vi "UHR-Fleezers Control (host) - 12.0.vi"() -> ()   [LabVIEW 2014] (continued)
  T41 = enum32{"Normal Display", "Dual Display (APD)", "FFT", "High Res Display"}
  T42 = cluster{"Origin Pixel":cluster{"X":sgl, "Y":sgl}, "Angle Relative to Horizontal (deg)":sgl, "Axis Reference":u32}
  T43 = typedef "Simple Grid Descriptor" = cluster{"X Step":sgl, "Y Step":sgl, "Unit":T44}
  T44 = typedef "Image Unit" = enum32{"Undefined", "Angström", "Micrometer", "Millimeter", "Centimeter", "Meter", "Kilometer", "Microinch", "Inch", "Feet", "Nautical miles", "Standard miles", "Steps"}
  T45 = cluster{"averaging mode":u16, "weighting mode":u16, "number of averages":u32}
  T46 = cluster{"dB On (F)":bool, "unwrap phase (F)":bool, "convert to degree (F)":bool}
  T47 = cluster{string, string, string, string, string, string, string, string}
  T48 = cluster{string, string, string, string, string, string, string, string, string, string, string, string}
  T49 = cluster{string, string, string, string, string, string, string, string, string, string, string, string, string}
  T50 = cluster{string, string, string, string, string, string, string, string, string, string, string, string, string, string}
  T51 = cluster{"BD 1 Frequency 1 (MHz)":dbl, "BD 1 Frequency 2 (MHz)":dbl}
  T52 = cluster{"f0":dbl, "df":dbl, "magnitude":dbl[]}[][]
diagram:
  w11 = T19 1073684535 items=["Service Request"=1073684491, "Trigger"=3221168138, "Clear"=1073684493, "VXI Signal"=1073684512, "VXI/VME Interrupt"=3221168161, "VXI/VME Sysfail"=1073684509, "VXI/VME Sysreset"=1073684510, "GPIB CIC"=1073684498, "GPIB Talk"=1073684499, "GPIB Listen"=1073684500, "PXI Interrupt"=1073684514, "Serial Break"=1073684515, "Serial TermChar"=1073684516, "Serial CTS"=1073684521, "Serial DSR"=1073684522, "Serial DCD"=1073684524, "Serial RI"=1073684526, "Serial Character"=1073684533, "USB Interrupt"=1073684535, "All Enabled"=1073709055] ("Event Type")
  w45 = 0.0 ("Total Volume\nFlowed P1 (uL)")
  w57 = u16 20 items=["1.0"=10, "1.5"=15, "2.0"=20] ("stop bits (10: 1 bit)")
  w60 = u16 20 items=["1.0"=10, "1.5"=15, "2.0"=20] ("stop bits (10: 1 bit)")
  w114 = u16 20 items=["1.0"=10, "1.5"=15, "2.0"=20] ("stop bits (10: 1 bit)")
  w121 = T20 2 items=["Grayscale (U8)", "Grayscale (I16)", "Grayscale (SGL)", "Complex (CSG)", "RGB (U32)", "HSL (U32)", "RGB (U64)", "Grayscale (U16)"] ("Image Type")
  w179 = cluster{"output high":i16, "output low":i16} {"output high"=3000, "output low"=0} ("FB output range 1")
  w250 = 10.0 ("y")
  w249 = 32767.0 ("y")
  w265 = 6.0  # clock mult.
  w266 = 49152000.0  # TCXO frequ.
  # "Open the RAW resource"
  # "Enable USB Interrupt Event"
  # "Safety limits on RF frequencies and amplitudes (for AOM protection)"
  # "Bottom 1 Harvard"
  # "Top 3 Harvard"
  # "Center Harvard"
  # "Bottom 1 Harvard"
  # "Top 3 Harvard"
  # "Center Harvard"
  n1 = Build Array("DIO count 1 (ticks)", "DIO count 2 (ticks)", "DIO count 3 (ticks)") -> (w166:u32[])
  n2 = local read "AO1"() -> (w244:dbl)
  n3 = local read "AO2"() -> (w243:dbl)
  n4 = local read "Scan Increment (MHz)"() -> (w261:dbl)
  n5 = local read "Continuous MCL Scanning"() -> (w231:bool)
  n6 = local read "Fast Scan Dir"() -> (w230:bool)
  n7 = local read "Number of scans (MCL)"() -> (w232:u64)
  n8 = property on="AI Count (ticks)" class="DigNum (strict)"("Val(Sgnl)"="AI Count (ticks)") -> ()  [unwired: 2 in, 2 out]
  n9 = Multiply(x=w244, y=w249) -> (x*y=w246:dbl)
  n10 = Multiply(x=w243, y=w249) -> (x*y=w248:dbl)
  n11 = Divide(x=w246, y=w250) -> (x/y=w245:dbl)
  n12 = Divide(x=w248, y=w250) -> (x/y=w247:dbl)
  n13 = To Word Integer(number=w245) -> (16bit integer=w242:i16)
  n14 = To Word Integer(number=w247) -> (16bit integer=w241:i16)
  n15 = Not(x=w230) -> (.not. x?=w225:bool)
  n16 = local read "Cycles/step (MCL)"() -> (w233:u64)
  n17 = Multiply(x=w261, y=1000.0) -> (x*y=w268:dbl)
  n18 = local read "Scan steps (MCL)"() -> (w234:u64)
  n19 = local write "Trap Pos FIFO Timeout"(u16 0 ("Trap Pos FIFO Timeout")) -> ()
  n20 = local read "Desired Scan Incr (V)"() -> (w236:dbl)
  n21 = Scale By Power Of 2(n=48, x=w268) -> (x*2^n=w269:dbl)
  n22 = Multiply(x=w266, y=w265) -> (x*y=w264:dbl)
  n23 = Divide(x=w269, y=w264) -> (x/y=w263:dbl)
  n24 = local read "Setpoints (V)"() -> (w280:cluster{"Set 1":dbl, "Set 2":dbl})
  n25 = To Quad Integer(1:w263) -> (0:w260:i64)
  n26 = Divide(x=40000000.0, y="AI Count (ticks)") -> (x/y=w221:dbl)
  n27 = Multiply(x=w236, y=32767.0) -> (x*y=w238:dbl)
  n28 = local read "Number Interlace Sets"() -> (w159:u8)
  n29 = Split 1D Array(array=w166, index=w159) -> (first subarray=w168:u32[])  [unwired: 1 out]
  n30 = Add Array Elements(numeric array=w168) -> (sum=w167:u32)
  n31 = local read "# Samples/channel"() -> (w253:u32)
  n32 = local read "Number of F/B Scans (AOD)"() -> (w254:u16)
  n33 = local read "Not-Interlacing Set"() -> (w158:enum32{"Set 1", "Set 2", "Set 3"})
  n34 = To Unsigned Byte Integer(number=w158) -> (unsigned 8bit integer=w164:u8)
  n35 = Index Array(array=w166, index=w164) -> (element=w165:u32)
  n36 = local read "Feedback On/Off"() -> (w283:cluster{"Set 1":bool, "Set 2":bool})
  n37 = local read "PID Gains"() -> (w275:T9)
  n38 = local read "Scan steps (AOD)"() -> (w259:u64)
  n39 = local read "All FB On/Off"() -> (w284:bool)
  n40 = local read "Cycles/step (AOD)"() -> (w258:u64)
  n41 = local write "AI rate (Hz)"(w221) -> ()
  n42 = Divide(x=w238, y=10.0) -> (x/y=w237:dbl)
  n43 = Multiply(x=w259, y=w258) -> (x*y=w257:u64)
  n44 = Multiply(x=3276.7, y=w280) -> (x*y=w279:cluster{"Set 1":dbl, "Set 2":dbl})
  n45 = To Word Integer(number=w237) -> (16bit integer=w235:i16)
  n46 = xnode "Open FPGA VI Reference"("resource name"=T21 "RIO1") -> ("FPGA VI Reference Out"=w43:T22, "error out"=w41:errorcluster)  [unwired: 1 in]
  n47 = Multiply(x=w257, y=u64 2) -> (x*y=w255:u64)
  n48 = local read "Sets to FIFO (Traps)"() -> (w287:T16)
  n49 = Divide(x=w221, y="FPGA Ave.") -> (x/y=w222:dbl)
  n50 = To Word Integer(number=w279) -> (16bit integer=w278:cluster{"Set 1":i16, "Set 2":i16})
  n51 = Unbundle By Name(w275) -> ("Set 1"=w274:T15, "Set 2"=w273:T15)
  n52 = Multiply(x=w255, y=w254) -> (x*y=w252:u64)
  n53 = local write "Ave. Rate (Hz)"(w222) -> ()
  n54 = Divide(x=w252, y=w253) -> (x/y=w251:dbl)
  n55 = Unbundle By Name(w278) -> ("Set 1"=w277:i16, "Set 2"=w276:i16)
  n56 = local read "2D or 1D Scan"() -> (w180:bool)
  n57 = local write "Data points/scans"(w252) -> ()
  n58 = local read "Scan BD"() -> (w270:bool)
  n59 = And(x=w283, y=w284) -> (x .and. y?=w282:cluster{"Set 1":bool, "Set 2":bool})
  n60 = local write "Data points/scan (f/b)"(w255) -> ()
  n61 = Reciprocal(x=w222) -> (1/x=w223:dbl)
  n62 = local read "N Acq Sets (Traps + Fl.)"() -> (w214:i16)
  n63 = local write "N sets should be saved"(w251) -> ()
  n64 = xnode "Invoke Method"("FPGA VI Reference In"=w43, "error in"=w41) -> ("FPGA VI Reference Out"=w178:T22, "error out"=w188:errorcluster)
  n65 = Unbundle By Name(w282) -> ("Set 1"=w286:bool, "Set 2"=w285:bool)
  n66 = local read "Interlace"() -> (w160:bool)
  n67 = Select(t=w167, s=w160, f=w165) -> (s? t:f=w157:u32)
  n68 = local write "Update Count (MCL)"(w157) -> ()
  n69 = local write "Total Counts (ticks)"(w157) -> ()
  n70 = local write "Ave. Period (s)"(w223) -> ()
  n71 = property on="2D or 1D Scan" class="Bool (strict)"("Val(Sgnl)"=w180) -> ()  [unwired: 2 in, 2 out]
  n72 = local read "APD Gate OFF Count"() -> (w84:u16)
  n73 = local read "Interlace OFF count"() -> (w87:u16)
  n74 = local read "Interlace ON count"() -> (w22:u16)
  n75 = local read "APD Gate ON Count"() -> (w80:u16)
  n76 = xnode "Read/Write Control"("FPGA VI Reference In"=w177, "error in"=w188, "ai count"="AI Count (ticks)", "Interlace ON/OFF"=w160, "Number Interlace Cycles"=w159, "AI1 Sets to FIFO"=w287, "FB On/Off Set 1"=w286, "FB On/Off Set 2"=w285, "Interlace Off Parameters"=w158, "FB Setpoint Set 1"=w277, "FB Setpoint Set 2"=w276, "FB Gains Set 1"=w274, "FB Gains Set 2"=w273, "FB output range 1"=w179, "FB output range 2"=w179, "Cycles per step"=w258, "Scan BD"=w270, "Number of scans"=w254, "Scan steps"=w259, "Scan freq.  increment"=w260, "AO1"=w242, "AO2"=w241, "Scan freq.  increment (MCL)"=w235, "Scan steps (MCL)"=w234, "Cycles per step (MCL)"=w233, "Number of scans (MCL)"=w232, "MCL count"=w157, "Cont. Scan (MCL)"=w231, "MCL Scan Axis"=w225, "1D or 2D Scan?"=w180, "N of AI1 Int Acq Sets"=w214, "Freq or Amp switch first"="Freq or Amp switch first", "Freq switch delay"="Freq switch delay", "Amp switch delay"="Amp switch delay", "Swap F1 and F2"="Swap F1 and F2", "APD to FIFO"=FALSE, "DIO count 1 (ticks)"="DIO count 1 (ticks)", "DIO count 2 (ticks)"="DIO count 2 (ticks)", "DIO count 3 (ticks)"="DIO count 3 (ticks)") -> ("FPGA VI Reference Out"=w91:T22, "error out"=w89:errorcluster)  [unwired: 1 in]
  n77 = local read "Duty frequency (ON 1/N cycles)"() -> (w86:u16)
  n78 = local read "APD Integration Time (s)"() -> (w72:dbl)
  n79 = local read "DMA Update Period (s)"() -> (w71:dbl)
  n80 = local read "Red Laser ON/Interlacing"() -> (w25:bool)
  n81 = Add(x=w80, y=w84) -> (x+y=w82:u16)
  n82 = local read "Laser interlacing mode (all lasers)"() -> (w24:enum32{"Laser ON", "Laser OFF", "Interlace"})
  n83 = Add(x=w22, y=w87) -> (x+y=w85:u16)
  n84 = local read "Green ON/Interlacing"() -> (w156:bool)
  n85 = Multiply(x=w82, y=w86) -> (x*y=w83:u16)
  n86 = Multiply(x="Red FB Setpoint (mV)", y=3.2767) -> (x*y=w15:dbl)
  n87 = Multiply(x=w86, y=w85) -> (x*y=w79:u16)
  n88 = Reciprocal(x=w72) -> (1/x=w69:dbl)
  n89 = Multiply(x=w72, y=40000000.0) -> (x*y=w68:dbl)
  n90 = Divide(x=w71, y=w72) -> (x/y=w74:dbl)
  n91 = Multiply(x="Green intensity % (FB OFF)", y=655.35) -> (x*y=w146:dbl)
  n92 = local read "Invert laser interlacing"() -> (w20:bool)
  n93 = case shown="False" w25 {
    tunnel: w24 -> [_ w311]
    tunnel: [enum32{"Laser ON", "Laser OFF", "Interlace"}."Laser OFF" ("Laser interlacing mode (all lasers)") w311] -> w23
    frame False {
    }
    frame True {
    }
  }
  n94 = local read "Invert APD Gate"() -> (w78:bool)
  n95 = Multiply(x="Green FB Setpoint (mV)", y=3.2767) -> (x*y=w143:dbl)
  n96 = local read "APD Gate"() -> (w77:enum32{"ON", "OFF", "Interlace"})
  n97 = Subtract(x=w83, y=w80) -> (x-y=w81:u16)
  n98 = To Word Integer(number=w15) -> (16bit integer=w14:i16)
  n99 = local write "Green FB Count"(w79) -> ()
  n100 = local write "APD Acq Rate (Hz)"(w69) -> ()
  n101 = To Unsigned Long Integer(number=w68) -> (unsigned 32bit integer=w66:u32)
  n102 = Multiply(x=2.0, y=w74) -> (x*y=w73:dbl)
  n103 = To Unsigned Word Integer(number=w146) -> (unsigned 16bit integer=w144:u16)
  n104 = Subtract(x=w79, y=w22) -> (x-y=w21:u16)
  n105 = local write "APD Samples/FIFO Acq."(w74) -> ()
  n106 = To Word Integer(number=w143) -> (16bit integer=w141:i16)
  n107 = local write "APD Elements/DMA read"(w73) -> ()
  n108 = case shown="False" w156 {
    tunnel: w24 -> [_ w313]
    tunnel: [enum32{"Laser ON", "Laser OFF", "Interlace"}."Laser OFF" ("Green laser mode") w313] -> w26
    frame False {
    }
    frame True {
    }
  }
  n109 = local write "APD Int. Count"(w66) -> ()
  n110 = Multiply(x="Red intensity % (FB OFF)", y=655.35) -> (x*y=w30:dbl)
  n111 = local read "Trap Pos. AI1 X Pre-scale"() -> (w101:u16)
  n112 = local read "Trap Pos FB Monitor\nT1 or T2"() -> (w108:bool)
  n113 = To Unsigned Word Integer(number=w30) -> (unsigned 16bit integer=w29:u16)
  n114 = local read "Trap Pos FB Int Count"() -> (w95:u16)
  n115 = local read "APD 1 AO Mult."() -> (w76:i16)
  n116 = local read "Trap Pos FB Negate Action"() -> (w107:bool)
  n117 = local read "APD 2 AO Mult."() -> (w75:i16)
  n118 = local read "Trap Pos. FB Offset Factor"() -> (w106:i64)
  n119 = local read "Trap Pos. FB Mult Factor"() -> (w105:i64)
  n120 = local read "Differential FB?"() -> (w63:bool)
  n121 = local read "Neg. TTrig FPGA"() -> (w65:bool)
  n122 = local read "Trap Pos. FB Gains"() -> (w103:T11)
  n123 = local read "Trap Pos. FB Range"() -> (w104:T12)
  n124 = xnode "Read/Write Control"("FPGA VI Reference In"=w91, "error in"=w89, "Invert APD Gate"=w78, "APD Gate ON Count"=w80, "APD Gate OFF Count"=w81, "APD Acq Rate Count"=w66, "APD Gate Operating Mode"=w77, "APD 1 AO scale factor"=w76, "APD 2 AO scale factor"=w75, "Green interlace ON count"=w22, "Green interlace OFF count"=w21, "Green interlace ON count 2"=w22, "Green interlace OFF count 2"=w21, "Green FB Count"=w79, "RI ON count"=w22, "RI OFF count"=w21) -> ("FPGA VI Reference Out"=w90:T22, "error out"=w88:errorcluster)
  n125 = xnode "Read/Write Control"("FPGA VI Reference In"=w90, "error in"=w88, "Invert GI 2"=w20, "Operating Mode 2"=w26, "Green FB Gains"="Green FB Gains", "Green FB Setpoint"=w141, "Green FB On/Off"="Green FB On/Off", "Current Out"=w144, "Green int current ON count adj"="Green int current ON count adj", "Operating Mode"=w26, "Invert GI"=w20, "Trap Pos FB Monitor T1 or T2"=w108, "Trap Pos FB Negate Action"=w107, "Trap Pos. FB Offset Factor"=w106, "Trap Pos. FB Mult Factor"=w105, "Trap Pos. FB Range"=w104, "Trap Pos. FB Gains"=w103, "Force feedback"=FALSE, "AI1 X Scale"=w101, "Trap Pos to FIFO"=TRUE, "Trap Pos FB Int Count"=w95, "TTrig Negate Pos"=w65, "FB Trig Integrate"="FB Trig Integrate", "Diff FB Measurement?"=w63, "Negate Diff?"="Negate Diff?", "RI Current Out"=w29, "Red operating mode"=w23, "RI operating mode 2"=w23, "Invert RI"=w20, "Invert RI 2"=w20, "Red FB Gains"="Red FB Gains", "Red FB On/Off"="Red FB On/Off", "Red FB Setpoint"=w14) -> ("FPGA VI Reference Out"=w154:T22, "error out"=w155:errorcluster)
  n126 = xnode "Invoke Method"("FPGA VI Reference In"=w154, "error in"=w155, "Requested Depth"="Trap AI FIFO Depth") -> ("FPGA VI Reference Out"=w110:T22, "error out"=w109:errorcluster)  [unwired: 1 out]
  n127 = xnode "Invoke Method"("FPGA VI Reference In"=w110, "error in"=w109, "Requested Depth"="Trap Position FIFO Depth") -> ("FPGA VI Reference Out"=w97:T22, "error out"=w96:errorcluster)  [unwired: 1 out]
  n128 = flat-sequence {
    tunnel: w178 -> [w318]
    tunnel: [w318] -> w177
    tunnel: [w317] -> w176
    tunnel: [w316] -> w175
    tunnel: [w314] -> w173
    tunnel: [w315] -> w174
    frame #0 {
      w315 = T17 {"Minimum"=0.0, "Maximum"=40.0, "Increment"=1.0} ("Min Max Inc")
      w314 = T17 {"Minimum"=0.0, "Maximum"=50.0, "Increment"=1.0} ("Data Entry Limits")
      w317 = T17 {"Minimum"=60.0, "Maximum"=90.0, "Increment"=1.0} ("Min Max Inc")
      w316 = T17 {"Minimum"=0.0, "Maximum"=50.0, "Increment"=1.0} ("Data Entry Limits")
      n129 = property on="BD 2 Frequency 1 (MHz)" class="DigNum (strict)"("Data Range"=w315) -> ()  [unwired: 2 in, 2 out]
      n130 = property on="BD 2 Frequency 3 (MHz)" class="DigNum (strict)"("Data Range"=w315) -> ()  [unwired: 2 in, 2 out]
      n131 = property on="BD 2 Frequency 2 (MHz)" class="DigNum (strict)"("Data Range"=w315) -> ()  [unwired: 2 in, 2 out]
      n132 = property on="BD 1 Frequency 1 (MHz)" class="DigNum (strict)"("Data Range"=w317) -> ()  [unwired: 2 in, 2 out]
      n133 = property on="BD 1 Frequency 2 (MHz)" class="DigNum (strict)"("Data Range"=w317) -> ()  [unwired: 2 in, 2 out]
      n134 = property on="BD 1 Frequency 3 (MHz)" class="DigNum (strict)"("Data Range"=w317) -> ()  [unwired: 2 in, 2 out]
      n135 = property on="BD 2 Amplitude 1 (%)" class="DigNum (strict)"("Data Range"=w314) -> ()  [unwired: 2 in, 2 out]
      n136 = property on="BD 2 Amplitude 2 (%)" class="DigNum (strict)"("Data Range"=w314) -> ()  [unwired: 2 in, 2 out]
      n137 = property on="BD 2 Amplitude 3 (%)" class="DigNum (strict)"("Data Range"=w314) -> ()  [unwired: 2 in, 2 out]
      n138 = property on="BD 1 Amplitude 3 (%)" class="DigNum (strict)"("Data Range"=w316) -> ()  [unwired: 2 in, 2 out]
      n139 = property on="BD 1 Amplitude 2 (%)" class="DigNum (strict)"("Data Range"=w316) -> ()  [unwired: 2 in, 2 out]
      n140 = property on="BD 1 Amplitude 1 (%)" class="DigNum (strict)"("Data Range"=w316) -> ()  [unwired: 2 in, 2 out]
      "X RF Frequency Limits (MHz)" <- w317
      "X RF Amplitude Limits (%)" <- w316
      "Y RF Amplitude Limits (%)" <- w314
      "Y RF Frequency Limits (MHz)" <- w315
    }
  }
  n141 = xnode "Invoke Method"("FPGA VI Reference In"=w97, "error in"=w96) -> ("FPGA VI Reference Out"=w187:T22, "error out"=w186:errorcluster)  [unwired: 1 in]
  n142 = flat-sequence "Initial FPGA Loop Relative Phase Adjustment" {
    tunnel: "Initial Phase Adjustment (APD 2 Gate)" -> [w321]
    tunnel: "Initial Phase Adjust (GI) 2" -> [w322]
    tunnel: "Initial Phase Adj. (MCL)" -> [w320]
    tunnel: w186 -> [w323]
    tunnel: w187 -> [w324]
    tunnel: "Initial Phase Adjust (GI)" -> [w325]
    tunnel: "Initial Phase Adjustment (AI1)" -> [w326]
    tunnel: [w326] -> w40
    tunnel: [w325] -> w39
    tunnel: [w324] -> w38
    tunnel: [w323] -> w37
    tunnel: [w320] -> w36
    tunnel: [w322] -> w35
    tunnel: [w321] -> w34
    tunnel: [w339] -> w196
    tunnel: [w333] -> w192
    tunnel: "Initial Phase Adjustment (APD Acq)" -> [w332]
    tunnel: "Initial Phase Adjustment (APD 1 Gate)" -> [w331]
    tunnel: "Initial Phase Adjust (Green FB)" -> [w330]
    tunnel: w40 -> [w338]
    tunnel: w39 -> [w337]
    tunnel: w38 -> [w336]
    tunnel: w37 -> [w335]
    tunnel: w36 -> [w334]
    tunnel: w35 -> [w329]
    tunnel: w34 -> [w328]
    tunnel: "Initial Phase Adjustment (RI)" -> [w327]
    tunnel: w196 -> [w341]
    tunnel: [w342] -> w193
    tunnel: w192 -> [w342]
    tunnel: [w341] -> w191
    tunnel: w193 -> [w345]
    tunnel: w191 -> [w344]
    tunnel: [w347] -> w190
    tunnel: [w346] -> w189
    tunnel: [w349] -> w194
    tunnel: [w350] -> w195
    tunnel: w190 -> [w350]
    tunnel: w189 -> [w349]
    frame #0 {
      n143 = Wait (ms)(milliseconds to wait=u32 100) -> ()  [unwired: 1 out]
    }
    frame #1 {
      n144 = xnode "Read/Write Control"("FPGA VI Reference In"=w336, "error in"=w335, "Phase count adjustment"=w338, "Phase count adjustment (GI)"=w337, "Phase count adjustment (MCL)"=w334, "Phase Count Adjustment (APD Acq)"=w332, "Phase count adjustment (APD 1 Gate)"=w331, "Phase count adjustment (APD 2 Gate)"=w328, "Phase count adjustment (Green FB)"=w330, "Phase count adjustment (GI) 2"=w329, "Phase count adjustment (RI)"=w327) -> ("FPGA VI Reference Out"=w333:T22, "error out"=w339:errorcluster)
    }
    frame #2 {
      n145 = Wait (ms)(milliseconds to wait=u32 100) -> ()  [unwired: 1 out]
    }
    frame #3 {
      w343 = TRUE
      n146 = xnode "Read/Write Control"("FPGA VI Reference In"=w345, "error in"=w344, "+ phase"=w343, "+ phase (GI)"=w343, "+ phase (MCL)"=w343, "+ phase (APD Acq)"=w343, "+ phase (APD 1 Gate)"=w343, "+ phase (APD 2 Gate)"=w343, "+ phase (Green FB)"=w343, "+ phase (GI) 2"=w343, "+ phase (RI)"=w343) -> ("FPGA VI Reference Out"=w346:T22, "error out"=w347:errorcluster)
    }
    frame #4 {
      n147 = Wait (ms)(milliseconds to wait=u32 100) -> ()  [unwired: 1 out]
    }
  }
  n148 = VISA Open(VISA resource name="USB port") -> (VISA resource name=w13:refnum<visa-resource-name>, error out=w12:errorcluster)  [unwired: 1 in, 3 out]
  n149 = local read "Phase adj. (Green FB)"() -> (w169:i16)
  n150 = local read "Phase adj. (GI) 2"() -> (w147:i16)
  n151 = local read "Phase adj. (RI)"() -> (w27:i16)
  n152 = local read "Phase adjust (MCL)"() -> (w226:i16)
  n153 = local read "Phase adj. (AI1)"() -> (w228:i16)
  n154 = local read "Phase adj. (GI)"() -> (w227:i16)
  n155 = VISA Enable Event(8:w12, 10:w11, 11:w13) -> (0:w8:errorcluster, 3:w7:refnum<visa-resource-name>)  [unwired: 1 out]
  n156 = xnode "Read/Write Control"("FPGA VI Reference In"=w194, "error in"=w195, "Phase count adjustment"=w228, "Phase count adjustment (GI)"=w227, "Phase count adjustment (MCL)"=w226, "Phase Count Adjustment (APD Acq)"="Phase Adj. (APD Acq)", "Phase count adjustment (APD 1 Gate)"="Phase Adj. (APD 1 Gate)", "Phase count adjustment (APD 2 Gate)"="Phase Adj. (APD 2 Gate)", "Phase count adjustment (Green FB)"=w169, "Phase count adjustment (GI) 2"=w147, "Phase count adjustment (RI)"=w27) -> ("FPGA VI Reference Out"=w42:T22, "error out"=w203:errorcluster)
  n157 = call "Initialize RF boards - interlace 3.vi"("error in"=w203, "FPGA VI Reference In"=w42) -> ("error out"=w201:errorcluster, "FPGA VI Reference Out"=w202:T22)
  n158 = call "set RF board frequency - interlace.vi"("Board 2 Frequency Limits"=w174, "Board 1 Frequency Limits"=w176, "error in"=w201, "FPGA VI Reference In"=w202, "Board 2 Frequency 3 (MHz)"="BD 2 Frequency 3 (MHz)", "Board 1 Frequency 3 (MHz)"="BD 1 Frequency 3 (MHz)", "Board 2 Frequency 2 (MHz)"="BD 2 Frequency 2 (MHz)", "Board 2 Frequency 1 (MHz)"="BD 2 Frequency 1 (MHz)", "Board 1 Frequency 2 (MHz)"="BD 1 Frequency 2 (MHz)", "Board 1 Frequency 1  (MHz)"="BD 1 Frequency 1 (MHz)") -> ("error out"=w302:errorcluster, "FPGA VI Reference Out"=w303:T22)
  n159 = call "set RF board amplitude - interlace.vi"("Board 2 Amplitude Limits"=w173, "Board 1 Amplitude Limits"=w175, "error in"=w302, "FPGA VI Reference In"=w303, "Board 2 Amplitude 3 (%)"="BD 2 Amplitude 3 (%)", "Board 1 Amplitude 3 (%)"="BD 1 Amplitude 3 (%)", "Board 2 Amplitude 2 (%)"="BD 2 Amplitude 2 (%)", "Board 2 Amplitude 1 (%)"="BD 2 Amplitude 1 (%)", "Board 1 Amplitude 2 (%)"="BD 1 Amplitude 2 (%)", "Board 1 Amplitude 1 (%)"="BD 1 Amplitude 1 (%)") -> ("error out"=w290:errorcluster, "FPGA VI Reference Out"=w291:T22)
  n160 = flat-sequence {
    tunnel: w291 -> [w360]
    tunnel: w290 -> [w359]
    tunnel: [w358] -> w295
    tunnel: [w357] -> w294
    tunnel: [w364] -> w293
    tunnel: w295 -> [w364]
    tunnel: [w363] -> w292
    tunnel: w294 -> [w363]
    tunnel: w293 -> [w373]
    tunnel: w292 -> [w372]
    tunnel: [w371] -> w51
    tunnel: [w370] -> w98
    frame #0 {
      w351 = FALSE ("Retract Pump 3")
      n161 = local read "Trap 1 (ON/OFF)"() -> (w352:bool)
      n162 = xnode "Read/Write Control"("FPGA VI Reference In"=w360, "error in"=w359, "Direct RF Box  Communication"=FALSE) -> ("FPGA VI Reference Out"=w358:T22, "error out"=w357:errorcluster)
      n163 = local write "Saving..."(FALSE ("Saving Data")) -> ()
      n164 = local write "Stop All"(FALSE ("Stop All")) -> ()
      n165 = local write "Retract Pump 1"(w351) -> ()
      n166 = local write "Retract Pump 3"(w351) -> ()
      n167 = local write "Index"(1.0 ("Index")) -> ()
      n168 = property on="Trap 1 ON" class="Bool (strict)"("Value"=w352) -> ()  [unwired: 2 in, 2 out]
      "Manipulating Trap" <- FALSE ("Manipulating Trap")
    }
    frame #1 {
      n169 = local read "Trap 2 (ON/OFF)"() -> (w362:bool)
      n170 = Wait (ms)(milliseconds to wait=u32 10) -> ()  [unwired: 1 out]
      n171 = property on="Trap 2 ON" class="Bool (strict)"("Val(Sgnl)"=w362) -> ()  [unwired: 2 in, 2 out]
    }
    frame #2 {
      n172 = local read "Scan Range (nm)"() -> (w366:dbl)
      n173 = xnode "Read/Write Control"("FPGA VI Reference In"=w373, "error in"=w372, "FPGA Controls  RF Box"=TRUE ("Direct RF Box  Communication")) -> ("FPGA VI Reference Out"=w371:T22, "error out"=w370:errorcluster)
      n174 = call "Update messages.vi"("Message to add"="UHR-Fleezers ready.", "Old message string"="") -> ("New message string"=w369:string)
      n175 = local write "Messages"(w369) -> ()
      n176 = property on="Scan Range (nm)" class="DigNum (strict)"("Val(Sgnl)"=w366) -> ()  [unwired: 2 in, 2 out]
    }
  }
  n177 = Subtract(x="BD 1 Frequency 1 (MHz)", y="BD 1 Frequency 2 (MHz)") -> (x-y=w213:dbl)
  n178 = Subtract(x="BD 2 Frequency 1 (MHz)", y="BD 2 Frequency 2 (MHz)") -> (x-y=w212:dbl)
  n179 = Square(x=w212) -> (x^2=w210:dbl)
  n180 = Square(x=w213) -> (x^2=w211:dbl)
  n181 = Add(x=w211, y=w210) -> (x+y=w209:dbl)
  n182 = Square Root(x=w209) -> (sqrt(x)=w208:dbl)
  n183 = local write "Trap D (MHz)"(w208) -> ()
  n184 = call "IMAQ Create"("Image Name"="APD 1 Image", "Image Type"=w121) -> ("New Image"=w120:T2)  [unwired: 3 in, 1 out]
  n185 = call "IMAQ Create"("Image Name"="APD 2 Image", "Image Type"=w121) -> ("New Image"=w119:T2)  [unwired: 3 in, 1 out]
  n186 = call "IMAQ Create"("Image Name"="Det. X Image", "Image Type"=w121) -> ("New Image"=w118:T2)  [unwired: 3 in, 1 out]
  n187 = call "IMAQ Create"("Image Name"="Det. Y Image", "Image Type"=w121) -> ("New Image"=w117:T2)  [unwired: 3 in, 1 out]
  n188 = Bundle("New Image"=w120, "New Image"=w119, "New Image"=w118, "New Image"=w117) -> (w116:T23)  [unwired: 1 in]
  n189 = call-poly "VISA Configure Serial Port"("VISA resource name"="Bottom  1 Harvard Syringe Pump Serial Port", "baud rate (9600)"=u32 115200, "stop bits (10: 1 bit)"=w57) -> ("VISA resource name out"=w53:refnum<visa-resource-name>, "error out"=w52:errorcluster)  [unwired: 4 in, 7 out]
  n190 = call-poly "VISA Configure Serial Port"("VISA resource name"="Top 3 Harvard Syringe Pump Serial Port", "baud rate (9600)"=u32 115200, "stop bits (10: 1 bit)"=w60) -> ("VISA resource name out"=w55:refnum<visa-resource-name>, "error out"=w54:errorcluster)  [unwired: 4 in, 7 out]
  n191 = call-poly "VISA Configure Serial Port"("VISA resource name"="Sample Chamber Stage Serial Port", "baud rate (9600)"=u32 19200) -> ("VISA resource name out"=w5:refnum<visa-resource-name>, "error out"=w130:errorcluster)  [unwired: 4 in, 8 out]
  "Stage Control Serial Error" <- w130
  n192 = while {
    shift-right: [w393] -> w4
    shift-left: w8 -> [w394]
    shift-right: [w391] -> w3
    shift-left: w7 -> [w392]
    tunnel: w5 -> [w390]
    stop <- w395 stop-if-true
    n193 = global read "FAST_Global_var.vi" "FAST L"() -> (→"FAST Z" →"FAST Z":bool)
    n194 = global read "FAST_Global_var.vi" "FAST R"() -> (→"FAST X-Y" →"FAST X-Y":bool)
    n195 = call "LogitechSubVi.vi"("USB port"=w392, "VISA resource name in 2 (for the Newport)"=w390, "error in (no error)"=w394, "X-Y Wait time"="XY Wait time", "Z Wait time"="Z Wait time", "XY Speed Definitions"="XY Speed Definitions", "Z Speed Definitions"="Z Speed Definitions") -> ("Right stick button"=→"Right stick button":bool, "Left stick button"=→"Left stick button":bool, "USB port out"=w391:refnum<visa-resource-name>, "error out"=w393:errorcluster, "A B X Y"=w380:cluster{"A":bool, "B":bool, "X":bool, "Y":bool}, "LB RB"=w389:T24, "U D L R"=w381:cluster{"U":bool, "D":bool, "L":bool, "R":bool}, "Sticks"=w388:T25)  [unwired: 5 in]
    n196 = Unbundle By Name(w381) -> ("U"=→"U":bool, "D"=→"D":bool, "L"=→"L":bool, "R"=→"R":bool)
    n197 = Unbundle By Name(w389) -> ("LB"=w379:bool, "RB"=w378:bool, "BACK"=w376:bool, "Logitech"=w375:bool, "START"=w377:bool)
    "LB" <- w378
    "RB" <- w379
    "BACK" <- w376
    "START" <- w377
    "Logitech" <- w375
    n198 = case shown="True" w378 {
      frame False {
      }
      frame True {
        n199 = local read "Trap 1 (ON/OFF)"() -> (w424:bool)
        n200 = Not(x=w424) -> (.not. x?=w425:bool)
        n201 = property on="Trap 1 (ON/OFF)" class="Bool (strict)"("Val(Sgnl)"=w425) -> ()  [unwired: 2 in, 2 out]
      }
    }
    n202 = case shown="True" w376 {
      selector: w376 -> [_ w420]
      frame False {
      }
      frame True {
        n203 = property on="Move to Position 1" class="Bool (strict)"("Val(Sgnl)"=w420) -> ()  [unwired: 2 in, 2 out]
      }
    }
    n204 = case shown="True" w375 {
      frame False {
      }
      frame True {
        n205 = local read "Sample Channel\nFlow"() -> (w419:bool)
        n206 = Not(x=w419) -> (.not. x?=w418:bool)
        n207 = property on="Sample Channel\nFlow" class="Bool (strict)"("Val(Sgnl)"=w418) -> ()  [unwired: 2 in, 2 out]
      }
    }
    n208 = case shown="True" w379 {
      frame False {
      }
      frame True {
        n209 = local read "Trap 2 (ON/OFF)"() -> (w422:bool)
        n210 = Not(x=w422) -> (.not. x?=w423:bool)
        n211 = property on="Trap 2 (ON/OFF)" class="Bool (strict)"("Val(Sgnl)"=w423) -> ()  [unwired: 2 in, 2 out]
      }
    }
    n212 = case shown="True" w377 {
      selector: w377 -> [_ w421]
      frame False {
      }
      frame True {
        n213 = property on="Move to Position 2" class="Bool (strict)"("Val(Sgnl)"=w421) -> ()  [unwired: 2 in, 2 out]
      }
    }
    n214 = Unbundle By Name(w388) -> ("Right X"=w415:i8, "Right Y"=w414:i8, "Left X"=w412:i8, "Left Y"=w410:i8)
    n215 = Not Equal To 0?(x=w415) -> (x != 0?=w417:bool)
    n216 = Not Equal To 0?(x=w410) -> (x != 0?=w411:bool)
    n217 = Not Equal To 0?(x=w412) -> (x != 0?=w413:bool)
    n218 = Unbundle By Name(w380) -> ("A"=w402:bool, "B"=w400:bool, "X"=w398:bool, "Y"=w396:bool)
    "B" <- w400
    "A" <- w402
    "Y" <- w396
    "X" <- w398
    n219 = case shown="\"Got ADig\", Default" "A command" {
      tunnel: w402 -> [w453 w455 w457 w460]
      frame "Got ADig", Default {
        n220 = case shown="True" w453 {
          selector: w453 -> [_ w454]
          frame False {
          }
          frame True {
            n221 = property on="Got ADig bead" class="Bool (strict)"("Val(Sgnl)"=w454) -> ()  [unwired: 2 in, 2 out]
          }
        }
      }
      frame "Dump" {
        n222 = case shown="True" w455 {
          selector: w455 -> [_ w456]
          frame False {
          }
          frame True {
            n223 = property on="Dump Beads" class="Bool (strict)"("Val(Sgnl)"=w456) -> ()  [unwired: 2 in, 2 out]
          }
        }
      }
      frame "Fish" {
        n224 = case shown="True" w457 {
          frame False {
          }
          frame True {
            n225 = local read "Fish"() -> (w458:bool)
            n226 = Not(x=w458) -> (.not. x?=w459:bool)
            n227 = property on="Fish" class="Bool (strict)"("Val(Sgnl)"=w459) -> ()  [unwired: 2 in, 2 out]
          }
        }
      }
      frame "Got DNA" {
        n228 = case shown="True" w460 {
          selector: w460 -> [_ w461]
          frame False {
          }
          frame True {
            n229 = property on="Got DNA bead" class="Bool (strict)"("Val(Sgnl)"=w461) -> ()  [unwired: 2 in, 2 out]
          }
        }
      }
    }
    n230 = case shown="\"Got DNA\", Default" "B command" {
      tunnel: w400 -> [w444 w446 w448 w450]
      frame "Got DNA", Default {
        n231 = case shown="True" w444 {
          selector: w444 -> [_ w445]
          frame False {
          }
          frame True {
            n232 = property on="Got DNA bead" class="Bool (strict)"("Val(Sgnl)"=w445) -> ()  [unwired: 2 in, 2 out]
          }
        }
      }
      frame "Got ADig" {
        n233 = case shown="True" w446 {
          selector: w446 -> [_ w447]
          frame False {
          }
          frame True {
            n234 = property on="Got ADig bead" class="Bool (strict)"("Val(Sgnl)"=w447) -> ()  [unwired: 2 in, 2 out]
          }
        }
      }
      frame "Dump" {
        n235 = case shown="True" w448 {
          selector: w448 -> [_ w449]
          frame False {
          }
          frame True {
            n236 = property on="Dump Beads" class="Bool (strict)"("Val(Sgnl)"=w449) -> ()  [unwired: 2 in, 2 out]
          }
        }
      }
      frame "Fish" {
        n237 = case shown="True" w450 {
          frame False {
          }
          frame True {
            n238 = local read "Fish"() -> (w451:bool)
            n239 = Not(x=w451) -> (.not. x?=w452:bool)
            n240 = property on="Fish" class="Bool (strict)"("Val(Sgnl)"=w452) -> ()  [unwired: 2 in, 2 out]
          }
        }
      }
    }
    n241 = Not Equal To 0?(x=w414) -> (x != 0?=w416:bool)
    n242 = case shown="True" w417 {
      tunnel: w415 -> [_ w465]
      frame False {
      }
      frame True {
        "Right X" <- w465
      }
    }
    n243 = case shown="True" w411 {
      tunnel: w410 -> [_ w462]
      frame False {
      }
      frame True {
        "Left Y" <- w462
      }
    }
    n244 = case shown="True" w416 {
      tunnel: w414 -> [_ w464]
      frame False {
      }
      frame True {
        "Right Y" <- w464
      }
    }
    n245 = case shown="\"Dump\", Default" "X command" {
      tunnel: w398 -> [w435 w437 w440 w442]
      frame "Dump", Default {
        n246 = case shown="True" w435 {
          selector: w435 -> [_ w436]
          frame False {
          }
          frame True {
            n247 = property on="Dump Beads" class="Bool (strict)"("Val(Sgnl)"=w436) -> ()  [unwired: 2 in, 2 out]
          }
        }
      }
      frame "Fish" {
        n248 = case shown="True" w437 {
          frame False {
          }
          frame True {
            n249 = local read "Fish"() -> (w438:bool)
            n250 = Not(x=w438) -> (.not. x?=w439:bool)
            n251 = property on="Fish" class="Bool (strict)"("Val(Sgnl)"=w439) -> ()  [unwired: 2 in, 2 out]
          }
        }
      }
      frame "Got ADig" {
        n252 = case shown="True" w440 {
          selector: w440 -> [_ w441]
          frame False {
          }
          frame True {
            n253 = property on="Got ADig bead" class="Bool (strict)"("Val(Sgnl)"=w441) -> ()  [unwired: 2 in, 2 out]
          }
        }
      }
      frame "Got DNA" {
        n254 = case shown="True" w442 {
          selector: w442 -> [_ w443]
          frame False {
          }
          frame True {
            n255 = property on="Got DNA bead" class="Bool (strict)"("Val(Sgnl)"=w443) -> ()  [unwired: 2 in, 2 out]
          }
        }
      }
    }
    n256 = case shown="True" w413 {
      tunnel: w412 -> [_ w463]
      frame False {
      }
      frame True {
        "Left X" <- w463
      }
    }
    n257 = case shown="\"Fish\", Default" "Y command" {
      tunnel: w396 -> [w426 w429 w431 w433]
      frame "Fish", Default {
        n258 = case shown="True" w426 {
          frame False {
          }
          frame True {
            n259 = local read "Fish"() -> (w427:bool)
            n260 = Not(x=w427) -> (.not. x?=w428:bool)
            n261 = property on="Fish" class="Bool (strict)"("Val(Sgnl)"=w428) -> ()  [unwired: 2 in, 2 out]
          }
        }
      }
      frame "Dump" {
        n262 = case shown="True" w429 {
          selector: w429 -> [_ w430]
          frame False {
          }
          frame True {
            n263 = property on="Dump Beads" class="Bool (strict)"("Val(Sgnl)"=w430) -> ()  [unwired: 2 in, 2 out]
          }
        }
      }
      frame "Got ADig" {
        n264 = case shown="True" w431 {
          selector: w431 -> [_ w432]
          frame False {
          }
          frame True {
            n265 = property on="Got ADig bead" class="Bool (strict)"("Val(Sgnl)"=w432) -> ()  [unwired: 2 in, 2 out]
          }
        }
      }
      frame "Got DNA" {
        n266 = case shown="True" w433 {
          selector: w433 -> [_ w434]
          frame False {
          }
          frame True {
            n267 = property on="Got DNA bead" class="Bool (strict)"("Val(Sgnl)"=w434) -> ()  [unwired: 2 in, 2 out]
          }
        }
      }
    }
    n268 = local read "Stop All"() -> (w395:bool)
  }
  n269 = VISA Close(VISA resource name=w3, error in (no error)=w4) -> (error out=w9:errorcluster)
  n270 = call <vilib>:"Simple Error Handler.vi"("error in (no error)"=w9) -> ()  [unwired: 1 in, 8 out]
  n271 = call-poly "VISA Configure Serial Port"("VISA resource name"="Center Harvard Syringe Pump Serial Port", "baud rate (9600)"=u32 115200, "stop bits (10: 1 bit)"=w114) -> ("VISA resource name out"=w111:refnum<visa-resource-name>, "error out"=w112:errorcluster)  [unwired: 4 in, 7 out]
  n272 = disable-structure shown="Disabled" {
    disable-tunnel: [w467 _] -> w272
    disable-tunnel: w51 -> [w466 _]
    frame Disabled {
      n273 = node-c288() -> (w469:T26)  [unwired: 4 out]
      n274 = timed-loop "Rough control of MCL mirror stage (debugging)" {
        tunnel: w466 -> [w472]
        tunnel: [w471] -> w467
        timing: w469 -> [_]
        timing-out: [_] -> w468
        stop <- w471 stop-if-true
        n275 = node-c288() -> ()  [unwired: 2 out]
        n276 = case shown="1" "MCL Mode" {
          tunnel: w472 -> [_ w475 w522]
          frame 0, Default {
          }
          frame 1 {
            n277 = node-c288() -> (w477:T26)  [unwired: 4 out]
            n278 = timed-loop "Oscillate MCL mirror" {
              timing: w477 -> [_]
              timing-out: [_] -> w476
              tunnel: w475 -> [w516]
              i -> [w515]
              stop <- w478 stop-if-true
              n279 = node-c288() -> (w514:i64)  [unwired: 1 out]
              n280 = Multiply(x="AO1", y=32767.0) -> (x*y=w510:dbl)
              n281 = Multiply(x="AO2", y=32767.0) -> (x*y=w505:dbl)
              n282 = Divide(x=w510, y=10.0) -> (x/y=w511:dbl)
              n283 = Divide(x=w505, y=10.0) -> (x/y=w506:dbl)
              n284 = To Word Integer(number=w511) -> (16bit integer=w503:i16)
              n285 = To Word Integer(number=w506) -> (16bit integer=w502:i16)
              n286 = Divide(x=w514, y=i64 1000) -> (x/y=w485:dbl)
              n287 = Multiply(x=w485, y=w515) -> (x*y=w496:dbl)
              n288 = Multiply(x="Osc. freq. (Hz) 2", y=6.283185307179586) -> (x*y=w497:dbl)
              n289 = Multiply(x=w497, y=w496) -> (x*y=w495:dbl)
              n290 = Sine(x=w495) -> (sin(x)=w494:dbl)
              n291 = Multiply(x=w494, y="Osc. amp. (V)") -> (x*y=w492:dbl)
              n292 = Add(x=w492, y="Osc. center (V)") -> (x+y=w490:dbl)
              n293 = Divide(x=w490, y=10.0) -> (x/y=w488:dbl)
              n294 = Multiply(x=w488, y=32767.0) -> (x*y=w483:dbl)
              n295 = Select(t=w483, s="Scan axis", f=w503) -> (s? t:f=w501:dbl)
              n296 = Select(t=w502, s="Scan axis", f=w483) -> (s? t:f=w500:dbl)
              n297 = local read "MCL Mode"() -> (w482:u16)
              n298 = Not Equal?(x=w482, y=u16 1) -> (x != y?=w479:bool)
              n299 = local read "Stop All"() -> (w480:bool)
              n300 = xnode "Read/Write Control"("FPGA VI Reference In"=w516, "AO1"=w501, "AO2"=w500) -> ()  [unwired: 1 in, 2 out]
              n301 = Compound Arithmetic op=OR(w480, w479) -> (w478:bool)
              n302 = node-c288() -> ()  [unwired: 2 out]
            }
            n303 = node-c288(w476) -> ()  [unwired: 1 out]
          }
          frame 2 {
            n304 = case shown="True" "Start Scan" {
              tunnel: w522 -> [_ w534]
              frame False {
              }
              frame True {
                n305 = Subtract(x="End (V)", y="Begin (V)") -> (x-y=w530:dbl)
                n306 = Decrement(x="N Points") -> (x-1=w529:dbl)
                n307 = Divide(x=w530, y=w529) -> (x/y=w527:dbl)
                n308 = for {
                  N: "N Points" -> [_]
                  tunnel: "Begin (V)" -> [w547]
                  tunnel: w534 -> [w539]
                  tunnel: [w538] -> w533 mode=indexing
                  tunnel: w527 -> [w537]
                  tunnel: [w535] -> w526 mode=indexing
                  i -> [w546]
                  n309 = Multiply(x=w537, y=w546) -> (x*y=w545:dbl)
                  n310 = Add(x=w547, y=w545) -> (x+y=w542:dbl)
                  n311 = local read "Scan axis"() -> (w536:bool)
                  n312 = local read "AO1"() -> (w544:dbl)
                  n313 = local read "AO2"() -> (w543:dbl)
                  n314 = Select(t=w542, s=w536, f=w544) -> (s? t:f=w541:dbl)
                  n315 = Select(t=w543, s=w536, f=w542) -> (s? t:f=w540:dbl)
                  n316 = flat-sequence {
                    tunnel: w541 -> [w551]
                    tunnel: w540 -> [w550]
                    tunnel: w539 -> [w548]
                    tunnel: [w561] -> w538
                    tunnel: [w560] -> w535
                    frame #0 {
                      w554 = 10.0 ("y")
                      w549 = 32767.0 ("y")
                      n317 = Multiply(x=w551, y=w549) -> (x*y=w557:dbl)
                      n318 = Multiply(x=w550, y=w549) -> (x*y=w555:dbl)
                      n319 = Divide(x=w557, y=w554) -> (x/y=w558:dbl)
                      n320 = Divide(x=w555, y=w554) -> (x/y=w556:dbl)
                      n321 = To Word Integer(number=w558) -> (16bit integer=w552:i16)
                      n322 = To Word Integer(number=w556) -> (16bit integer=w553:i16)
                      n323 = xnode "Read/Write Control"("FPGA VI Reference In"=w548, "AO1"=w552, "AO2"=w553) -> ()  [unwired: 1 in, 2 out]
                    }
                    frame #1 {
                      n324 = Wait (ms)(milliseconds to wait="DAQ Delay (ms)") -> ()  [unwired: 1 out]
                    }
                    frame #2 {
                      n325 = local read "Slow mean"() -> (w561:dbl)
                      n326 = local read "Sigma"() -> (w560:dbl)
                    }
                  }
                }
                n327 = Bundle("Begin (V)"="Begin (V)", w527, w533) -> (→"MCL Scan":cluster{"Begin (V)":dbl, dbl, dbl[]})  [unwired: 1 out]
                n328 = Bundle("Begin (V)"="Begin (V)", w527, w526) -> (→"MCL Scan 2":cluster{"Begin (V)":dbl, dbl, dbl[]})  [unwired: 1 out]
              }
            }
          }
        }
        n329 = local read "Stop All"() -> (w471:bool)
        n330 = node-c288() -> ()  [unwired: 2 out]
      }
      n331 = node-c288(w468) -> ()  [unwired: 1 out]
    }
    frame Enabled {
    }
  }
  n332 = node-c288(3 ("Processor")) -> (w135:T26)  [unwired: 3 out]
  n333 = timed-loop "Oscillate Trap/AOM (fishing, debugging)" {
    tunnel: w51 -> [w565]
    tunnel: [w564] -> w140
    timing: w135 -> [_]
    timing-out: [_] -> w134
    stop <- w564 stop-if-true
    n334 = node-c288() -> ()  [unwired: 2 out]
    n335 = event shown="[0] \"Oscillate Set 1\", \"Fish\": Value Change" {
      selector: _ -> [_ _ _]
      dyn-events: _ -> [_ _ _]
      timeout: _ -> [_ _ _]
      tunnel: w565 -> [w572 _ _]
      tunnel: [FALSE ("Stop All") _ w1257] -> w564
      event "Oscillate Set 1", "Fish": Value Change {
        n336 = event-data() -> ()  [unwired: 6 out]
        n337 = local read "Oscillate Set 1"() -> (w571:bool)
        n338 = Or(x=w571, y="Fish") -> (x .or. y?=w569:bool)
        n339 = case shown="True" w569 {
          tunnel: w572 -> [_ w575]
          tunnel: "Fish" -> [_ w573]
          frame False {
          }
          frame True {
            n340 = case shown="True" w573 {
              selector: w573 -> [w578 w579]
              tunnel: [w578 w579] -> w574
              frame False {
              }
              frame True {
                w580 = FALSE ("Tether")
                n341 = local write "Scan axis 2"(TRUE) -> ()
                n342 = local write "Tether"(w580) -> ()
                n343 = local write "Hysteresis"(w580) -> ()
                n344 = local write "Multiple tether"(w580) -> ()
                n345 = local write "Bad fit"(w580) -> ()
                n346 = local write "Good tether"(w580) -> ()
                n347 = property on="Trap D (MHz)" class="DigNum (strict)"("Val(Sgnl)"="Furthest D (MHz)") -> ()  [unwired: 2 in, 2 out]
                n348 = local read "Flow ON\nduring cal?"() -> (w581:bool)
                n349 = Or(x="Flow ON during \nfishing?", y=w581) -> (x .or. y?=w582:bool)
                n350 = Wait (ms)(milliseconds to wait=u32 500) -> ()  [unwired: 1 out]
                n351 = property on="Sample Channel\nFlow" class="Bool (strict)"("Val(Sgnl)"=w582) -> ()  [unwired: 2 in, 2 out]
              }
            }
            n352 = node-c288() -> (w577:T26)  [unwired: 4 out]
            n353 = timed-loop "Oscillate AOD" {
              timing: w577 -> [_]
              timing-out: [_] -> w576
              tunnel: w575 -> [w594]
              tunnel: w574 -> [w588]
              i -> [w596]
              stop <- w587 stop-if-true
              n354 = node-c288() -> (w595:i64)  [unwired: 1 out]
              n355 = flat-sequence {
                tunnel: w596 -> [w623]
                tunnel: w595 -> [w622]
                tunnel: w594 -> [w601]
                tunnel: w588 -> [w604]
                tunnel: [w604] -> w593
                tunnel: [w603] -> w592
                tunnel: [w600] -> w591
                tunnel: [w597] -> w589
                tunnel: w593 -> [w666]
                tunnel: w592 -> [w664]
                tunnel: w591 -> [w663]
                tunnel: [w662] -> w590
                tunnel: w589 -> [w661]
                tunnel: [w822] -> w587
                tunnel: w590 -> [w821]
                frame #0 {
                  n356 = Divide(x=w622, y=i64 1000) -> (x/y=w617:dbl)
                  n357 = Multiply(x=w617, y=w623) -> (x*y=w619:dbl)
                  n358 = local read "BD 1 Frequency 2 (MHz)"() -> (w602:dbl)
                  n359 = Multiply(x="Osc. freq. (Hz)", y=6.283185307179586) -> (x*y=w620:dbl)
                  n360 = Multiply(x=w620, y=w619) -> (x*y=w599:dbl)
                  n361 = local read "BD 1 Frequency 1 (MHz)"() -> (w607:dbl)
                  n362 = local read "BD 2 Frequency 1 (MHz)"() -> (w606:dbl)
                  n363 = case shown="True" w604 {
                    tunnel: w599 -> [w629 w634]
                    tunnel: w607 -> [_ w645]
                    tunnel: w602 -> [_ w646]
                    tunnel: [w626 w640] -> w605
                    tunnel: [FALSE w637] -> w600
                    tunnel: [0.0 w630] -> w597
                    frame False {
                      n364 = Sine(x=w629) -> (sin(x)=w627:dbl)
                      n365 = Multiply(x=w627, y="Osc. amp. (MHz)") -> (x*y=w626:dbl)
                    }
                    frame True {
                      n366 = Cosine(x=w634) -> (cos(x)=w649:dbl)
                      n367 = Subtract(x=w646, y=w645) -> (x-y=w644:dbl)
                      n368 = Decrement(x=w649) -> (x-1=w648:dbl)
                      n369 = Subtract(x=w644, y="Closest D (MHz)") -> (x-y=w641:dbl)
                      n370 = Divide(x=w648, y=-2.0) -> (x/y=w642:dbl)
                      n371 = Multiply(x=w642, y=w641) -> (x*y=w640:dbl)
                      n372 = local read "Vec Mean of T1 T2"() -> (w636:dbl[])
                      n373 = Greater?(x=w636, y="Stop F (pN)") -> (0:w638:bool[])
                      n374 = Or Array Elements(Boolean array=w638) -> (logical OR=w637:bool)
                      n375 = Divide(x=w634, y=6.283185307179586) -> (x/y=w633:dbl)
                      n376 = Round Toward +Infinity(x=w633) -> (ceil(x): smallest int >= x=w630:dbl)
                      "Attempts" <- w630
                      n377 = Greater?(x=w630, y="Attempt Limit") -> (0:w632:bool)
                      n378 = case shown="True" w632 {
                        frame False {
                        }
                        frame True {
                          n379 = local write "Fish"(FALSE ("Fish for Tether")) -> ()
                          n380 = local read "Messages"() -> (w651:string)
                          n381 = flat-sequence {
                            frame #0 {
                              n382 = call <vilib>:"Beep.vi"("use system alert? (T)"=FALSE, "duration (msec)"=u32 200, "frequency (Hz)"=u32 500) -> ()  [unwired: 9 out]
                            }
                            frame #1 {
                              n383 = Wait (ms)(milliseconds to wait=u32 100) -> ()  [unwired: 1 out]
                            }
                            frame #2 {
                              n384 = call <vilib>:"Beep.vi"("use system alert? (T)"=FALSE, "duration (msec)"=u32 200, "frequency (Hz)"=u32 500) -> ()  [unwired: 9 in]
                            }
                          }
                          n385 = call "Update messages.vi"("Message to add"="Tether fishing timeout." ("Messages"), "Old message string"=w651) -> ("New message string"=→"Messages":string)
                        }
                      }
                    }
                  }
                  n386 = Select(t=w607, s="Scan axis 2", f=w606) -> (s? t:f=w610:dbl)
                  n387 = Add(x=w605, y=w610) -> (x+y=w603:dbl)
                  n388 = Select(t=w603, s="Scan axis 2", f=w607) -> (s? t:f=w613:dbl)
                  n389 = Select(t=w606, s="Scan axis 2", f=w603) -> (s? t:f=w612:dbl)
                  n390 = local read "Y RF Frequency Limits (MHz)"() -> (w608:T17)
                  n391 = local read "X RF Frequency Limits (MHz)"() -> (w609:T17)
                  n392 = local read "BD 2 Frequency 2 (MHz)"() -> (w615:dbl)
                  n393 = local read "BD 2 Frequency 3 (MHz)"() -> (w614:dbl)
                  n394 = local read "BD 1 Frequency 3 (MHz)"() -> (w616:dbl)
                  n395 = call "set RF board frequency - interlace.vi"("Board 2 Frequency Limits"=w608, "Board 1 Frequency Limits"=w609, "FPGA VI Reference In"=w601, "Board 2 Frequency 3 (MHz)"=w614, "Board 1 Frequency 3 (MHz)"=w616, "Board 2 Frequency 2 (MHz)"=w615, "Board 2 Frequency 1 (MHz)"=w612, "Board 1 Frequency 2 (MHz)"=w602, "Board 1 Frequency 1  (MHz)"=w613) -> ()  [unwired: 1 in, 2 out]
                }
                frame #1 {
                  n396 = And(x=w666, y=w663) -> (x .and. y?=w665:bool)
                  n397 = case "Only if were fishing and now formed tether" shown="True" w665 {
                    tunnel: w664 -> [w668 w683]
                    tunnel: [w667 w682] -> w662
                    tunnel: w661 -> [_ w678]
                    frame False {
                      n398 = local read "Fish"() -> (w667:bool)
                      n399 = case shown="False" w667 {
                        tunnel: w668 -> [w669 _]
                        frame False {
                          n400 = property on="BD 1 Frequency 1 (MHz)" class="DigNum (strict)"("Val(Sgnl)"=w669) -> ()  [unwired: 2 in, 2 out]
                        }
                        frame True {
                        }
                      }
                    }
                    frame True {
                      w682 = FALSE ("Fish for Tether")
                      n401 = call <vilib>:"Beep.vi"() -> ()  [unwired: 3 in, 9 out]
                      n402 = Number To Decimal String(number=w678, width (-)=i16 1) -> (decimal integer string=w676:string)
                      n403 = Concatenate Strings("Formed tether in ", w676, " attempt(s)." ("string")) -> (w673:string)
                      n404 = local read "Messages"() -> (w680:string)
                      n405 = local write "Fish"(w682) -> ()
                      n406 = call "Update messages.vi"("Message to add"=w673, "Old message string"=w680) -> ("New message string"=w679:string)
                      n407 = local write "Messages"(w679) -> ()
                      n408 = Get Date/Time In Seconds() -> (seconds since 1Jan1904=→"Time tether formed":timestamp)
                      n409 = local read "Flow ON\nduring cal?"() -> (w670:bool)
                      n410 = property on="Sample Channel\nFlow" class="Bool (strict)"("Val(Sgnl)"=w670) -> (error out=w671:errorcluster)  [unwired: 2 in, 1 out]
                      n411 = case shown="\"2\", \"3\", \"4\", \"5\", \"6\"" "Then..." {
                        selector: "Then..." -> [_ w686 _ _]
                        tunnel: w683 -> [w685 _ _ _]
                        tunnel: w671 -> [_ _ _ _]
                        frame "1", Default {
                          n412 = property on="BD 1 Frequency 1 (MHz)" class="DigNum (strict)"("Val(Sgnl)"=w685) -> ()  [unwired: 2 in, 2 out]
                        }
                        frame "2", "3", "4", "5", "6" {
                          n413 = flat-sequence {
                            tunnel: w686 -> [w692]
                            frame #0 {
                              n414 = local read "Flow ON\nduring cal?"() -> (w687:bool)
                              n415 = property on="Sample Channel\nFlow" class="Bool (strict)"("Val(Sgnl)"=w687) -> ()  [unwired: 2 in, 2 out]
                              n416 = property on="Trap D (MHz)" class="DigNum (strict)"("Val(Sgnl)"="Move to D 1 (MHz)") -> ()  [unwired: 2 in, 2 out]
                            }
                            frame #1 {
                              n417 = local read "Wait Before Save (s)"() -> (w689:u32)
                              n418 = Multiply(x=u32 1000 ("milliseconds to wait"), y=w689) -> (x*y=w691:u32)
                              n419 = Wait (ms)(milliseconds to wait=w691) -> ()  [unwired: 1 out]
                            }
                            frame #2 {
                              n420 = case shown="\"5\", \"6\"" w692 {
                                selector: w692 -> [w695 w705 _]
                                frame "3", "4" {
                                n421 = flat-sequence {
                                tunnel: w695 -> [w696]
                                tunnel: [w696] -> w693
                                tunnel: [w698] -> w694
                                tunnel: w693 -> [w698]
                                tunnel: w694 -> [w702]
                                frame #0 {
                                n422 = property on="Green ON/Interlacing" class="Bool (strict)"("Val(Sgnl)"=TRUE ("Value (Signaling)")) -> ()  [unwired: 2 in, 2 out]
                                }
                                frame #1 {
                                n423 = Multiply(x="Wait Before Save (s)", y=u32 1000 ("x")) -> (x*y=w700:u32)
                                n424 = Wait (ms)(milliseconds to wait=w700) -> ()  [unwired: 1 out]
                                }
                                frame #2 {
                                n425 = property on="Start Saving" class="Bool (strict)"("Value"=TRUE ("Start Saving")) -> ()  [unwired: 2 in, 2 out]
                                n426 = case shown="\"4\"" w702 {
                                frame Default {
                                }
                                frame "4" {
                                n427 = property on="Fl. Triggered..." class="Bool (strict)"("Val(Sgnl)"=TRUE ("Value (Signaling)")) -> ()  [unwired: 2 in, 2 out]
                                }
                                }
                                }
                                }
                                }
                                frame "5", "6" {
                                n428 = stacked-sequence {
                                tunnel: w705 -> [_ _ _ _ _ _ w717]
                                frame #0 {
                                n429 = Replace Array Subset(array=u32[] [0] ("Index Values"), new element="Raster Set\nUpon Tether", index=0) -> (w706:u32[])
                                n430 = property on="Saved AOD Raster Scan Parameter Sets" class="Arr (strict)"("Index Values"=w706) -> ()  [unwired: 2 in, 2 out]
                                }
                                frame #1 {
                                n431 = Wait (ms)(milliseconds to wait=u32 500) -> ()  [unwired: 1 out]
                                }